vi "TLB Native Dynamic Events ver 0.26c.vi"() -> ()   [LabVIEW 2018] (continued)
                n641 = case shown="True" w1877 {
                  tunnel: [w1886 w1892] -> w1882
                  tunnel: w1878 -> [w1884 w1890]
                  frame False {
                    n642 = for {
                      tunnel: string[] ["CLOSE CLAW", "START TIMER"] ("element") -> [w1887] mode=indexing
                      shift-right: [w1889] -> w1886
                      shift-left: w1884 -> [w1888]
                      n643 = Enqueue Element(queue=w1888, element=w1887) -> (queue out=w1889:refnum<queue>)  [unwired: 2 in, 2 out]
                    }
                  }
                  frame True {
                    n644 = for {
                      shift-right: [w1894] -> w1892
                      shift-left: w1890 -> [w1895]
                      tunnel: string[] ["READ STEPPER VALUES", "", ""] -> [w1893] mode=indexing
                      n645 = Enqueue Element(queue=w1895, element=w1893) -> (queue out=w1894:refnum<queue>)  [unwired: 2 in, 2 out]
                    }
                  }
                }
                n646 = Or(x=w1877, y=w1873) -> (x .or. y?=w1880:bool)
                n647 = Select(t=State_Type_Definitions,_for_0.26g_versions_and_later_2."True Stop" ("Enum"), s=w1873, f=State_Type_Definitions,_for_0.26g_versions_and_later_2."Task 8K: RAISE MY SWORD" ("Enum")) -> (s? t:f=w1875:T18)
                n648 = Select(t=w1875, s=w1880, f=State_Type_Definitions,_for_0.26g_versions_and_later_2."Task 8J: CLOSE CLAW" ("Enum")) -> (s? t:f=w1879:T18)
              }
              frame "Exit" {
                n649 = for {
                  shift-right: [w1902] -> w1899
                  shift-left: w1896 -> [w1903]
                  tunnel: string[] ["STOP", "RESET ENCODERS", "RESET YAW", "ARDUINO MODE 0"] -> [w1901] mode=indexing
                  n650 = Enqueue Element(queue=w1903, element=w1901) -> (queue out=w1902:refnum<queue>)  [unwired: 2 in, 2 out]
                }
              }
            }
          }
          frame 37 {
            # ">>> yStepper command>>>"
            # ">> Manual override >>"
            n651 = Dequeue Element(queue=w1914, timeout in ms (-1)=w1913, error in (no error)=w1915) -> (element=w1912:T10)  [unwired: 3 out]
            n652 = Equal?(x=w1911, y=u8 60) -> (x = y?=w1909:bool)
            n653 = case shown="\"Start Task 1\", Default" w1912 {
              tunnel: [w1925 State_Type_Definitions,_for_0.26g_versions_and_later_2."True Stop" ("Enum")] -> w1916
              tunnel: [w1928 w1945] -> w1917
              tunnel: [State_Type_Definitions,_for_0.26g_versions_and_later_2."Idle" ("Enum") State_Type_Definitions,_for_0.26g_versions_and_later_2."Shutdown" ("Enum")] -> w1918
              tunnel: w1909 -> [w1924 _]
              tunnel: w1908 -> [w1923 _]
              tunnel: w1907 -> [w1919 w1942]
              frame "Start Task 1", Default {
                # "Stays in Task 5_A until stepper reaches desired \nheight"
                # "T: Go back to idle, F: Continue with task\""
                # ">> Manual override >>"
                n654 = case shown="True" w1924 {
                  tunnel: [w1932 w1938] -> w1928
                  tunnel: w1919 -> [w1930 w1936]
                  frame False {
                    n655 = for {
                      tunnel: string[] ["Z STEPPER CAM HEIGHT", "READ STEPPER VALUES"] ("element") -> [w1933] mode=indexing
                      shift-right: [w1935] -> w1932
                      shift-left: w1930 -> [w1934]
                      n656 = Enqueue Element(queue=w1934, element=w1933) -> (queue out=w1935:refnum<queue>)  [unwired: 2 in, 2 out]
                    }
                  }
                  frame True {
                    n657 = for {
                      shift-right: [w1940] -> w1938
                      shift-left: w1936 -> [w1941]
                      tunnel: string[] ["CAM CLOSE", "DISPOSE CAM BUFFERS", "DISPOSE PROC BUFFERS", "RESET ENCODERS"] -> [w1939] mode=indexing
                      n658 = Enqueue Element(queue=w1941, element=w1939) -> (queue out=w1940:refnum<queue>)  [unwired: 2 in, 2 out]
                    }
                  }
                }
                n659 = Or(x=w1924, y=w1923) -> (x .or. y?=w1926:bool)
                n660 = Select(t=State_Type_Definitions,_for_0.26g_versions_and_later_2."True Stop" ("Enum"), s=w1923, f=State_Type_Definitions,_for_0.26g_versions_and_later_2."True Stop" ("Enum")) -> (s? t:f=w1920:T18)
                n661 = Select(t=w1920, s=w1926, f=State_Type_Definitions,_for_0.26g_versions_and_later_2."Task 8K: RAISE MY SWORD" ("Enum")) -> (s? t:f=w1925:T18)
              }
              frame "Exit" {
                n662 = for {
                  shift-right: [w1948] -> w1945
                  shift-left: w1942 -> [w1949]
                  tunnel: string[] ["STOP", "RESET ENCODERS", "RESET YAW", "ARDUINO MODE 0"] -> [w1947] mode=indexing
                  n663 = Enqueue Element(queue=w1949, element=w1947) -> (queue out=w1948:refnum<queue>)  [unwired: 2 in, 2 out]
                }
              }
            }
          }
          frame 38 {
            # ">>> Motor control cluster >>>"
            # ">> Stepper height reeached >>"
            # ">>> yStepper command>>>"
            # ">> Manual override >>"
            n664 = Dequeue Element(queue=w1961, timeout in ms (-1)=w1956, error in (no error)=w1960) -> (element=w1964:T10)  [unwired: 3 out]
            n665 = Equal?(x=w1958, y=u8 40) -> (x = y?=w1962:bool)
            n666 = case shown="\"Start Task 1\", Default" w1964 {
              tunnel: [w1975 State_Type_Definitions,_for_0.26g_versions_and_later_2."True Stop" ("Enum")] -> w1954
              tunnel: [w1973 w1990] -> w1953
              tunnel: w1957 -> [w1972 _]
              tunnel: w1959 -> [w1966 _]
              tunnel: [State_Type_Definitions,_for_0.26g_versions_and_later_2."Idle" ("Enum") State_Type_Definitions,_for_0.26g_versions_and_later_2."Shutdown" ("Enum")] -> w1955
              tunnel: w1962 -> [w1965 _]
              frame "Start Task 1", Default {
                # ">> WIill proceed to part ii if not manual override >>"
                # ">>If ENABLE or Trigger is set to true>>"
                n667 = Or(x=w1965, y=w1966) -> (x .or. y?=w1967:bool)
                n668 = case shown="True" w1965 {
                  tunnel: [w1978 w1984] -> w1973
                  tunnel: w1972 -> [w1977 w1983]
                  frame False {
                    n669 = for {
                      shift-right: [w1980] -> w1978
                      shift-left: w1977 -> [w1981]
                      tunnel: string[] ["Z STEPPER BOX HEIGHT", "READ STEPPER VALUES"] ("element") -> [w1979] mode=indexing
                      n670 = Enqueue Element(queue=w1981, element=w1979) -> (queue out=w1980:refnum<queue>)  [unwired: 2 in, 2 out]
                    }
                  }
                  frame True {
                    n671 = for {
                      shift-right: [w1986] -> w1984
                      shift-left: w1983 -> [w1987]
                      tunnel: string[] ["OPEN LIFE CAM", "SET TIMER 5", "", "", "", ""] -> [w1985] mode=indexing
                      n672 = Enqueue Element(queue=w1987, element=w1985) -> (queue out=w1986:refnum<queue>)  [unwired: 2 in, 2 out]
                    }
                  }
                }
                n673 = Select(t=State_Type_Definitions,_for_0.26g_versions_and_later_2."True Stop" ("Enum"), s=w1966, f=State_Type_Definitions."Task 9F: SCAN IMAGE" ("Enum")) -> (s? t:f=w1969:u16)
                n674 = Select(t=w1969, s=w1967, f=State_Type_Definitions,_for_0.26g_versions_and_later_2."Task 9A: Raise Arm" ("Enum")) -> (s? t:f=w1975:u16)
              }
              frame "Exit" {
                n675 = for {
                  shift-right: [w1993] -> w1990
                  shift-left: _ -> [w1994]
                  tunnel: string[] ["STOP", "RESET ENCODERS", "RESET YAW", ""] -> [w1992] mode=indexing
                  n676 = Enqueue Element(queue=w1994, element=w1992) -> (queue out=w1993:refnum<queue>)  [unwired: 2 in, 2 out]
                }
              }
            }
          }
          frame 39 {
            # ">>> Motor control cluster >>>"
            # ">>> yStepper command>>>"
            n677 = Dequeue Element(queue=w2008, timeout in ms (-1)=w2007, error in (no error)=w2006) -> (element=w2010:T10)  [unwired: 3 out]
            n678 = In Range and Coerce(upper limit=65.0, x=w2000, lower limit=58.0) -> (In Range?=w1997:bool)  [unwired: 1 out]
            n679 = case shown="\"Start Task 1\", Default" w2010 {
              tunnel: w2001 -> [w2013 _]
              tunnel: [w2021 State_Type_Definitions,_for_0.26g_versions_and_later_2."True Stop" ("Enum")] -> w2003
              tunnel: w2009 -> [w2019 w2037]
              tunnel: [w2018 w2036] -> w2002
              tunnel: [State_Type_Definitions,_for_0.26g_versions_and_later_2."Idle" ("Enum") State_Type_Definitions,_for_0.26g_versions_and_later_2."Shutdown" ("Enum")] -> w2004
              tunnel: w1997 -> [w2011 _]
              frame "Start Task 1", Default {
                n680 = Or(x=w2011, y=w2013) -> (x .or. y?=w2012:bool)
                n681 = case shown="True" w2011 {
                  tunnel: w2019 -> [w2024 w2030]
                  tunnel: [w2023 w2028] -> w2018
                  frame False {
                    n682 = for {
                      shift-right: [w2026] -> w2023
                      shift-left: w2024 -> [w2027]
                      tunnel: string[] ["READ NAVX", "R-CW", "READ ULTRASONIC"] ("element") -> [w2025] mode=indexing
                      n683 = Enqueue Element(queue=w2027, element=w2025) -> (queue out=w2026:refnum<queue>)  [unwired: 2 in, 2 out]
                    }
                  }
                  frame True {
                    n684 = for {
                      shift-right: [w2032] -> w2028
                      shift-left: w2030 -> [w2033]
                      tunnel: string[] ["STOP", "RESET ENCODERS", "RESET YAW", "ARDUINO - ULTRASONIC", ""] -> [w2031] mode=indexing
                      n685 = Enqueue Element(queue=w2033, element=w2031) -> (queue out=w2032:refnum<queue>)  [unwired: 2 in, 2 out]
                    }
                  }
                }
                n686 = Select(t=State_Type_Definitions,_for_0.26g_versions_and_later_2."True Stop" ("Enum"), s=w2013, f=State_Type_Definitions,_for_0.26g_versions_and_later_2."Task 9C: Detect Box") -> (s? t:f=w2015:T18)
                n687 = Select(t=w2015, s=w2012, f=State_Type_Definitions,_for_0.26g_versions_and_later_2."Task 9B: Rotate to Angle" ("Enum")) -> (s? t:f=w2021:T18)
              }
              frame "Exit" {
                n688 = for {
                  shift-right: [w2040] -> w2036
                  shift-left: w2037 -> [w2041]
                  tunnel: string[] ["STOP", "RESET ENCODERS", "RESET YAW", ""] -> [w2039] mode=indexing
                  n689 = Enqueue Element(queue=w2041, element=w2039) -> (queue out=w2040:refnum<queue>)  [unwired: 2 in, 2 out]
                }
              }
            }
          }
          frame 40 {
            # ">>> Motor control cluster >>>"
            # ">>Line Detected>>"
            # ">>Action Queue>>"
            # ">>> yStepper command>>>"
            n690 = Dequeue Element(queue=w2053, timeout in ms (-1)=w2052, error in (no error)=w2051) -> (element=w2054:T10)  [unwired: 3 out]
            n691 = case shown="\"Start Task 1\", Default" w2054 {
              tunnel: w2049 -> [w2055 _]
              tunnel: [w2065 State_Type_Definitions,_for_0.26g_versions_and_later_2."True Stop" ("Enum")] -> w2046
              tunnel: w2050 -> [w2063 w2081]
              tunnel: [w2062 w2080] -> w2045
              tunnel: [State_Type_Definitions,_for_0.26g_versions_and_later_2."Idle" ("Enum") State_Type_Definitions,_for_0.26g_versions_and_later_2."Shutdown" ("Enum")] -> w2048
              tunnel: w2043 -> [w2056 _]
              frame "Start Task 1", Default {
                n692 = Or(x=w2055, y=w2056) -> (x .or. y?=w2057:bool)
                n693 = case shown="True" w2056 {
                  tunnel: w2063 -> [w2068 w2074]
                  tunnel: [w2067 w2072] -> w2062
                  frame False {
                    n694 = for {
                      shift-right: [w2070] -> w2067
                      shift-left: w2068 -> [w2071]
                      tunnel: string[] ["READ IR", "READ LINE SENSOR", "FORWARD - IR ASSIST"] ("element") -> [w2069] mode=indexing
                      n695 = Enqueue Element(queue=w2071, element=w2069) -> (queue out=w2070:refnum<queue>)  [unwired: 2 in, 2 out]
                    }
                  }
                  frame True {
                    n696 = for {
                      shift-right: [w2076] -> w2072
                      shift-left: w2074 -> [w2077]
                      tunnel: string[] ["STOP", "RESET ENCODERS", "RESET YAW", ""] -> [w2075] mode=indexing
                      n697 = Enqueue Element(queue=w2077, element=w2075) -> (queue out=w2076:refnum<queue>)  [unwired: 2 in, 2 out]
                    }
                  }
                }
                n698 = Select(t=State_Type_Definitions,_for_0.26g_versions_and_later_2."True Stop" ("Enum"), s=w2055, f=State_Type_Definitions,_for_0.26g_versions_and_later_2."Task 9D: MOVE FORWARD") -> (s? t:f=w2059:T18)
                n699 = Select(t=w2059, s=w2057, f=State_Type_Definitions,_for_0.26g_versions_and_later_2."Task 9C: Detect Box" ("Enum")) -> (s? t:f=w2065:T18)
              }
              frame "Exit" {
                n700 = for {
                  shift-right: [w2084] -> w2080
                  shift-left: w2081 -> [w2085]
                  tunnel: string[] ["STOP", "RESET ENCODERS", "RESET YAW", ""] -> [w2083] mode=indexing
                  n701 = Enqueue Element(queue=w2085, element=w2083) -> (queue out=w2084:refnum<queue>)  [unwired: 2 in, 2 out]
                }
              }
            }
          }
          frame 41 {
            (unwired) 50.0 ("y")
            # ">> Item Selection Bias >>"
            # ">> Wall detected >>"
            # ">> Manual override >>"
            # ">>Table Detected>>"
            # ">>> Motor control cluster >>>"
            # ">>Table or wall detectected>>"
            # ">>Action Queue>>"
            # ">>> yStepper command>>>"
            n702 = Dequeue Element(queue=w2103, timeout in ms (-1)=w2102, error in (no error)=w2101) -> (element=w2104:T10)  [unwired: 3 out]
            n703 = Less Or Equal?(x=w2092, y=20.0) -> (x <= y?=w2087:bool)
            n704 = Less?(x=w2090, y=20.0) -> (x < y?=w2088:bool)
            n705 = Or(x=w2087, y=w2088) -> (x .or. y?=w2086:bool)
            n706 = case shown="\"Start Task 1\", Default" w2104 {
              tunnel: w2099 -> [w2105 _]
              tunnel: [w2115 State_Type_Definitions,_for_0.26g_versions_and_later_2."True Stop" ("Enum")] -> w2096
              tunnel: w2100 -> [w2113 w2131]
              tunnel: [w2112 w2130] -> w2095
              tunnel: [State_Type_Definitions,_for_0.26g_versions_and_later_2."Idle" ("Enum") State_Type_Definitions,_for_0.26g_versions_and_later_2."Shutdown" ("Enum")] -> w2098
              tunnel: w2086 -> [w2106 _]
              frame "Start Task 1", Default {
                n707 = Or(x=w2105, y=w2106) -> (x .or. y?=w2107:bool)
                n708 = case shown="True" w2106 {
                  tunnel: w2113 -> [w2118 w2124]
                  tunnel: [w2117 w2122] -> w2112
                  frame False {
                    n709 = for {
                      shift-right: [w2120] -> w2117
                      shift-left: w2118 -> [w2121]
                      tunnel: string[] ["READ IR", "FORWARD - IR ASSIST", "READ ULTRASONIC"] ("element") -> [w2119] mode=indexing
                      n710 = Enqueue Element(queue=w2121, element=w2119) -> (queue out=w2120:refnum<queue>)  [unwired: 2 in, 2 out]
                    }
                  }
                  frame True {
                    n711 = for {
                      shift-right: [w2126] -> w2122
                      shift-left: w2124 -> [w2127]
                      tunnel: string[] ["STOP", "RESET ENCODERS", "RESET YAW", ""] -> [w2125] mode=indexing
                      n712 = Enqueue Element(queue=w2127, element=w2125) -> (queue out=w2126:refnum<queue>)  [unwired: 2 in, 2 out]
                    }
                  }
                }
                n713 = Select(t=State_Type_Definitions,_for_0.26g_versions_and_later_2."True Stop" ("Enum"), s=w2105, f=State_Type_Definitions,_for_0.26g_versions_and_later_2."Task 9E: MOVE LEFT") -> (s? t:f=w2109:T18)
                n714 = Select(t=w2109, s=w2107, f=State_Type_Definitions,_for_0.26g_versions_and_later_2."Task 9D: MOVE FORWARD" ("Enum")) -> (s? t:f=w2115:T18)
              }
              frame "Exit" {
                n715 = for {
                  shift-right: [w2134] -> w2130
                  shift-left: w2131 -> [w2135]
                  tunnel: string[] ["STOP", "RESET ENCODERS", "RESET YAW", ""] -> [w2133] mode=indexing
                  n716 = Enqueue Element(queue=w2135, element=w2133) -> (queue out=w2134:refnum<queue>)  [unwired: 2 in, 2 out]
                }
              }
            }
          }
          frame 42 {
            # ">> Item Selection Bias >>"
            # ">> Line detected? >>"
            # ">> Manual override >>"
            # ">>> Motor control cluster >>>"
            # ">>Action Queue>>"
            # ">>> yStepper command>>>"
            n717 = Dequeue Element(queue=w2147, timeout in ms (-1)=w2146, error in (no error)=w2145) -> (element=w2148:T10)  [unwired: 3 out]
            n718 = case shown="\"Start Task 1\", Default" w2148 {
              tunnel: w2143 -> [w2149 _]
              tunnel: [w2159 State_Type_Definitions,_for_0.26g_versions_and_later_2."True Stop" ("Enum")] -> w2140
              tunnel: w2144 -> [w2157 w2175]
              tunnel: [w2156 w2174] -> w2139
              tunnel: [State_Type_Definitions,_for_0.26g_versions_and_later_2."Idle" ("Enum") State_Type_Definitions,_for_0.26g_versions_and_later_2."Shutdown" ("Enum")] -> w2142
              tunnel: w2136 -> [w2150 _]
              frame "Start Task 1", Default {
                n719 = Or(x=w2149, y=w2150) -> (x .or. y?=w2151:bool)
                n720 = case shown="True" w2150 {
                  tunnel: w2157 -> [w2162 w2168]
                  tunnel: [w2161 w2166] -> w2156
                  frame False {
                    n721 = for {
                      shift-right: [w2164] -> w2161
                      shift-left: w2162 -> [w2165]
                      tunnel: string[] ["LEFT", "READ NAVX", "READ LINE SENSOR", ""] ("element") -> [w2163] mode=indexing
                      n722 = Enqueue Element(queue=w2165, element=w2163) -> (queue out=w2164:refnum<queue>)  [unwired: 2 in, 2 out]
                    }
                  }
                  frame True {
                    n723 = for {
                      shift-right: [w2170] -> w2166
                      shift-left: w2168 -> [w2171]
                      tunnel: string[] ["STOP", "RESET ENCODERS", "RESET YAW", "RESET FLAGS", "OPEN LIFE CAM", "SET TIMER 2"] -> [w2169] mode=indexing
                      n724 = Enqueue Element(queue=w2171, element=w2169) -> (queue out=w2170:refnum<queue>)  [unwired: 2 in, 2 out]
                    }
                  }
                }
                n725 = Select(t=State_Type_Definitions,_for_0.26g_versions_and_later_2."True Stop" ("Enum"), s=w2149, f=State_Type_Definitions."Task 9F: SCAN IMAGE") -> (s? t:f=w2153:u16)
                n726 = Select(t=w2153, s=w2151, f=State_Type_Definitions,_for_0.26g_versions_and_later_2."Task 9E: MOVE LEFT" ("Enum")) -> (s? t:f=w2159:u16)
              }
              frame "Exit" {
                n727 = for {
                  shift-right: [w2178] -> w2174
                  shift-left: w2175 -> [w2179]
                  tunnel: string[] ["STOP", "RESET ENCODERS", "RESET YAW", ""] -> [w2177] mode=indexing
                  n728 = Enqueue Element(queue=w2179, element=w2177) -> (queue out=w2178:refnum<queue>)  [unwired: 2 in, 2 out]
                }
              }
            }
          }
          frame 43 {
            # ">>> Motor control cluster >>>"
            # ">>Time up? >>"
            # ">>> yStepper command>>>"
            # ">> Manual override >>"
            n729 = Dequeue Element(queue=w2191, timeout in ms (-1)=w2187, error in (no error)=w2190) -> (element=w2192:T10)  [unwired: 3 out]
            n730 = case shown="\"Start Task 1\", Default" w2192 {
              tunnel: [w2203 State_Type_Definitions,_for_0.26g_versions_and_later_2."True Stop" ("Enum")] -> w2185
              tunnel: [w2201 w2219] -> w2184
              tunnel: w2188 -> [w2200 w2216]
              tunnel: w2189 -> [w2194 _]
              tunnel: [State_Type_Definitions,_for_0.26g_versions_and_later_2."Idle" ("Enum") State_Type_Definitions,_for_0.26g_versions_and_later_2."Shutdown" ("Enum")] -> w2186
              tunnel: w2180 -> [w2193 _]
              frame "Start Task 1", Default {
                # ">> WIill proceed to part ii if not manual override >>"
                # ">>If ENABLE or Trigger is set to true>>"
                n731 = Or(x=w2193, y=w2194) -> (x .or. y?=w2195:bool)
                n732 = case shown="True" w2193 {
                  tunnel: [w2206 w2212] -> w2201
                  tunnel: w2200 -> [w2205 w2211]
                  frame False {
                    n733 = for {
                      shift-right: [w2208] -> w2206
                      shift-left: w2205 -> [w2209]
                      tunnel: string[] ["CAM ACQ", "START TIMER"] ("element") -> [w2207] mode=indexing
                      n734 = Enqueue Element(queue=w2209, element=w2207) -> (queue out=w2208:refnum<queue>)  [unwired: 2 in, 2 out]
                    }
                  }
                  frame True {
                    n735 = for {
                      shift-right: [w2214] -> w2212
                      shift-left: w2211 -> [w2215]
                      tunnel: string[] ["CLOSE CAM", "SET TIMER 2", "RESET FLAGS", "", "", ""] -> [w2213] mode=indexing
                      n736 = Enqueue Element(queue=w2215, element=w2213) -> (queue out=w2214:refnum<queue>)  [unwired: 2 in, 2 out]
                    }
                  }
                }
                n737 = Select(t=State_Type_Definitions,_for_0.26g_versions_and_later_2."True Stop" ("Enum"), s=w2194, f=State_Type_Definitions."Task 9G: PROCESS COLOUR" ("Enum")) -> (s? t:f=w2197:u16)
                n738 = Select(t=w2197, s=w2195, f=State_Type_Definitions."Task 9F: SCAN IMAGE" ("Enum")) -> (s? t:f=w2203:u16)
              }
              frame "Exit" {
                n739 = for {
                  shift-right: [w2222] -> w2219
                  shift-left: w2216 -> [w2223]
                  tunnel: string[] ["STOP", "RESET ENCODERS", "RESET YAW", ""] -> [w2221] mode=indexing
                  n740 = Enqueue Element(queue=w2223, element=w2221) -> (queue out=w2222:refnum<queue>)  [unwired: 2 in, 2 out]
                }
              }
            }
          }
          frame 44 {
            # ">>> Motor control cluster >>>"
            # ">>> yStepper command>>>"
            n741 = Dequeue Element(queue=w2231, timeout in ms (-1)=w2230, error in (no error)=w2229) -> (element=w2236:T10)  [unwired: 3 out]
            n742 = case shown="\"Start Task 1\", Default" w2236 {
              tunnel: w2224 -> [w2239 _]
              tunnel: [w2246 State_Type_Definitions,_for_0.26g_versions_and_later_2."True Stop" ("Enum")] -> w2235
              tunnel: w2228 -> [w2238 _]
              tunnel: w2232 -> [w2245 w2262]
              tunnel: [w2244 w2263] -> w2234
              tunnel: [State_Type_Definitions,_for_0.26g_versions_and_later_2."Idle" ("Enum") State_Type_Definitions,_for_0.26g_versions_and_later_2."Shutdown" ("Enum")] -> w2233
              frame "Start Task 1", Default {
                n743 = case shown="False" w2239 {
                  tunnel: w2245 -> [w2249 w2256]
                  tunnel: [w2250 w2255] -> w2244
                  frame False {
                    n744 = for {
                      tunnel: string[] ["START TIMER", "COLOUR PROCESSING", ""] ("element") -> [w2251] mode=indexing
                      shift-right: [w2253] -> w2250
                      shift-left: w2249 -> [w2252]
                      n745 = Enqueue Element(queue=w2252, element=w2251) -> (queue out=w2253:refnum<queue>)  [unwired: 2 in, 2 out]
                    }
                  }
                  frame True {
                    n746 = for {
                      shift-right: [w2258] -> w2255
                      shift-left: w2256 -> [w2259]
                      tunnel: string[] ["DISPOSE BUFFERS", "CLOSE CAM", "RESET ENCODERS", "RESET YAW", "RESET FLAGS"] -> [w2257] mode=indexing
                      n747 = Enqueue Element(queue=w2259, element=w2257) -> (queue out=w2258:refnum<queue>)  [unwired: 2 in, 2 out]
                    }
                  }
                }
                n748 = Or(x=w2239, y=w2238) -> (x .or. y?=w2237:bool)
                n749 = Select(t=State_Type_Definitions,_for_0.26g_versions_and_later_2."True Stop" ("Enum"), s=w2238, f=State_Type_Definitions,_for_0.26g_versions_and_later_2."True Stop" ("Enum")) -> (s? t:f=w2240:T18)
                n750 = Select(t=w2240, s=w2237, f=State_Type_Definitions."Task 9G: PROCESS COLOUR" ("Enum")) -> (s? t:f=w2246:u16)
              }
              frame "Exit" {
                n751 = for {
                  shift-right: [w2266] -> w2263
                  shift-left: w2262 -> [w2267]
                  tunnel: string[] ["STOP", "RESET ENCODERS", "RESET YAW", "ARDUINO MODE 0"] -> [w2265] mode=indexing
                  n752 = Enqueue Element(queue=w2267, element=w2265) -> (queue out=w2266:refnum<queue>)  [unwired: 2 in, 2 out]
                }
              }
            }
          }
          frame 45 {
            # ">> Item Selection Bias >>"
            # ">>> Motor control cluster >>>"
            # ">>> yStepper command>>>"
            n753 = Dequeue Element(queue=w2277, timeout in ms (-1)=w2278, error in (no error)=w2279) -> (element=w2281:T10)  [unwired: 3 out]
            n754 = Greater?(x=w2269, y=50.0) -> (0:w2270:bool)
            n755 = And(x=w2271, y=w2270) -> (x .and. y?=w2272:bool)
            n756 = case shown="\"Start Task 1\", Default" w2281 {
              tunnel: w2272 -> [w2287 _]
              tunnel: [w2294 State_Type_Definitions,_for_0.26g_versions_and_later_2."True Stop" ("Enum")] -> w2274
              tunnel: w2280 -> [w2286 _]
              tunnel: w2276 -> [w2293 w2310]
              tunnel: [w2292 w2311] -> w2275
              tunnel: [State_Type_Definitions,_for_0.26g_versions_and_later_2."Idle" ("Enum") State_Type_Definitions,_for_0.26g_versions_and_later_2."Shutdown" ("Enum")] -> w2273
              frame "Start Task 1", Default {
                n757 = case shown="True" w2287 {
                  tunnel: w2293 -> [w2297 w2304]
                  tunnel: [w2298 w2303] -> w2292
                  frame False {
                    n758 = for {
                      tunnel: string[] ["READ LINE SENSOR", "READ NAVX", "RIGHT", "READ ENCODERS"] ("element") -> [w2299] mode=indexing
                      shift-right: [w2301] -> w2298
                      shift-left: w2297 -> [w2300]
                      n759 = Enqueue Element(queue=w2300, element=w2299) -> (queue out=w2301:refnum<queue>)  [unwired: 2 in, 2 out]
                    }
                  }
                  frame True {
                    n760 = for {
                      shift-right: [w2306] -> w2303
                      shift-left: w2304 -> [w2307]
                      tunnel: string[] ["STOP", "RESET ENCODERS", "RESET YAW", "OPEN LIFE CAM", "SET TIMER 5", "RESET FLAGS"] -> [w2305] mode=indexing
                      n761 = Enqueue Element(queue=w2307, element=w2305) -> (queue out=w2306:refnum<queue>)  [unwired: 2 in, 2 out]
                    }
                  }
                }
                n762 = Or(x=w2287, y=w2286) -> (x .or. y?=w2285:bool)
                n763 = Select(t=State_Type_Definitions,_for_0.26g_versions_and_later_2."True Stop" ("Enum"), s=w2286, f=State_Type_Definitions,_for_0.26d_versions_and_later."Task 9I: SCAN IMAGE" ("Enum")) -> (s? t:f=w2288:u16)
                n764 = Select(t=w2288, s=w2285, f=State_Type_Definitions."Task 9H: MOVE RIGHT" ("Enum")) -> (s? t:f=w2294:u16)
              }
              frame "Exit" {
                n765 = for {
                  shift-right: [w2314] -> w2311
                  shift-left: w2310 -> [w2315]
                  tunnel: string[] ["STOP", "RESET ENCODERS", "RESET YAW", "ARDUINO MODE 0"] -> [w2313] mode=indexing
                  n766 = Enqueue Element(queue=w2315, element=w2313) -> (queue out=w2314:refnum<queue>)  [unwired: 2 in, 2 out]
                }
              }
            }
          }
          frame 46 {
            # ">> Item Selection Bias >>"
            n767 = Dequeue Element(queue=w2317, timeout in ms (-1)=w2318, error in (no error)=w2319) -> (element=w2325:T10)  [unwired: 3 out]
            n768 = case shown="\"Start Task 1\", Default" w2325 {
              tunnel: w2316 -> [w2331 _]
              tunnel: [w2338 State_Type_Definitions,_for_0.26g_versions_and_later_2."True Stop" ("Enum")] -> w2322
              tunnel: w2320 -> [w2330 _]
              tunnel: w2324 -> [w2337 w2354]
              tunnel: [w2336 w2355] -> w2323
              tunnel: [State_Type_Definitions,_for_0.26g_versions_and_later_2."Idle" ("Enum") State_Type_Definitions,_for_0.26g_versions_and_later_2."Shutdown" ("Enum")] -> w2321
              frame "Start Task 1", Default {
                n769 = case shown="True" w2331 {
                  tunnel: w2337 -> [w2341 w2348]
                  tunnel: [w2342 w2347] -> w2336
                  frame False {
                    n770 = for {
                      tunnel: string[] ["START TIMER", "CAM ACQ", ""] ("element") -> [w2343] mode=indexing
                      shift-right: [w2345] -> w2342
                      shift-left: w2341 -> [w2344]
                      n771 = Enqueue Element(queue=w2344, element=w2343) -> (queue out=w2345:refnum<queue>)  [unwired: 2 in, 2 out]
                    }
                  }
                  frame True {
                    n772 = for {
                      shift-right: [w2350] -> w2347
                      shift-left: w2348 -> [w2351]
                      tunnel: string[] ["CLOSE CAM", "SET TIMER 5", "", "", "", ""] -> [w2349] mode=indexing
                      n773 = Enqueue Element(queue=w2351, element=w2349) -> (queue out=w2350:refnum<queue>)  [unwired: 2 in, 2 out]
                    }
                  }
                }
                n774 = Or(x=w2331, y=w2330) -> (x .or. y?=w2329:bool)
                n775 = Select(t=State_Type_Definitions,_for_0.26g_versions_and_later_2."True Stop" ("Enum"), s=w2330, f=State_Type_Definitions,_for_0.26d_versions_and_later."Task 9J: PROCESS COLOUR" ("Enum")) -> (s? t:f=w2332:u16)
                n776 = Select(t=w2332, s=w2329, f=State_Type_Definitions,_for_0.26d_versions_and_later."Task 9I: SCAN IMAGE" ("Enum")) -> (s? t:f=w2338:u16)
              }
              frame "Exit" {
                n777 = for {
                  shift-right: [w2358] -> w2355
                  shift-left: w2354 -> [w2359]
                  tunnel: string[] ["STOP", "RESET ENCODERS", "RESET YAW", "ARDUINO MODE 0"] -> [w2357] mode=indexing
                  n778 = Enqueue Element(queue=w2359, element=w2357) -> (queue out=w2358:refnum<queue>)  [unwired: 2 in, 2 out]
                }
              }
            }
          }
          frame 47 {
            # ">> Item Selection Bias >>"
            n779 = Dequeue Element(queue=w2365, timeout in ms (-1)=w2366, error in (no error)=w2367) -> (element=w2369:T10)  [unwired: 3 out]
            n780 = case shown="\"Start Task 1\", Default" w2369 {
              tunnel: w2360 -> [w2375 _]
              tunnel: [w2382 State_Type_Definitions,_for_0.26g_versions_and_later_2."True Stop" ("Enum")] -> w2363
              tunnel: w2368 -> [w2374 _]
              tunnel: w2364 -> [w2381 w2398]
              tunnel: [w2380 w2399] -> w2362
              tunnel: [State_Type_Definitions,_for_0.26g_versions_and_later_2."Idle" ("Enum") State_Type_Definitions,_for_0.26g_versions_and_later_2."Shutdown" ("Enum")] -> w2361
              frame "Start Task 1", Default {
                n781 = case shown="True" w2375 {
                  tunnel: w2381 -> [w2385 w2392]
                  tunnel: [w2386 w2391] -> w2380
                  frame False {
                    n782 = for {
                      tunnel: string[] ["START TIMER", "COLOUR PROCESSING", ""] ("element") -> [w2387] mode=indexing
                      shift-right: [w2389] -> w2386
                      shift-left: w2385 -> [w2388]
                      n783 = Enqueue Element(queue=w2388, element=w2387) -> (queue out=w2389:refnum<queue>)  [unwired: 2 in, 2 out]
                    }
                  }
                  frame True {
                    n784 = for {
                      shift-right: [w2394] -> w2391
                      shift-left: w2392 -> [w2395]
                      tunnel: string[] ["CLOSE CAM", "DISPOSE BUFFERS", "RESET ENCODERS", "RESET YAW", "RESET FLAGS", ""] -> [w2393] mode=indexing
                      n785 = Enqueue Element(queue=w2395, element=w2393) -> (queue out=w2394:refnum<queue>)  [unwired: 2 in, 2 out]
                    }
                  }
                }
                n786 = Or(x=w2375, y=w2374) -> (x .or. y?=w2373:bool)
                n787 = Select(t=State_Type_Definitions,_for_0.26g_versions_and_later_2."True Stop" ("Enum"), s=w2374, f=State_Type_Definitions,_for_0.26g_versions_and_later_2."True Stop" ("Enum")) -> (s? t:f=w2376:T18)
                n788 = Select(t=w2376, s=w2373, f=State_Type_Definitions,_for_0.26d_versions_and_later."Task 9J: PROCESS COLOUR" ("Enum")) -> (s? t:f=w2382:u16)
              }
              frame "Exit" {
                n789 = for {
                  shift-right: [w2402] -> w2399
                  shift-left: w2398 -> [w2403]
                  tunnel: string[] ["STOP", "RESET ENCODERS", "RESET YAW", "ARDUINO MODE 0"] -> [w2401] mode=indexing
                  n790 = Enqueue Element(queue=w2403, element=w2401) -> (queue out=w2402:refnum<queue>)  [unwired: 2 in, 2 out]
                }
              }
            }
          }
          frame 48 {
            # ">>> Motor control cluster >>>"
            # ">>> yStepper command>>>"
            # ">> Item Selection Bias >>"
            n791 = Less?(x=w2407, y=-38.0) -> (x < y?=w2405:bool)
            n792 = Dequeue Element(queue=w2413, timeout in ms (-1)=w2412, error in (no error)=w2411) -> (element=w2415:T10)  [unwired: 3 out]
            n793 = case shown="\"Start Task 1\", Default" w2415 {
              tunnel: w2405 -> [w2421 _]
              tunnel: [w2428 State_Type_Definitions,_for_0.26g_versions_and_later_2."True Stop" ("Enum")] -> w2409
              tunnel: w2410 -> [w2420 _]
              tunnel: w2414 -> [w2427 w2444]
              tunnel: [w2426 w2445] -> w2404
              tunnel: [State_Type_Definitions,_for_0.26g_versions_and_later_2."Idle" ("Enum") State_Type_Definitions,_for_0.26g_versions_and_later_2."Shutdown" ("Enum")] -> w2408
              frame "Start Task 1", Default {
                n794 = case shown="True" w2421 {
                  tunnel: w2427 -> [w2431 w2438]
                  tunnel: [w2432 w2437] -> w2426
                  frame False {
                    n795 = for {
                      tunnel: string[] ["READ ENCODERS", "R-CW"] ("element") -> [w2433] mode=indexing
                      shift-right: [w2435] -> w2432
                      shift-left: w2431 -> [w2434]
                      n796 = Enqueue Element(queue=w2434, element=w2433) -> (queue out=w2435:refnum<queue>)  [unwired: 2 in, 2 out]
                    }
                  }
                  frame True {
                    n797 = for {
                      shift-right: [w2440] -> w2437
                      shift-left: w2438 -> [w2441]
                      tunnel: string[] ["STOP", "RESET ENCODERS", "RESET FLAGS", "RESET YAW", "READ IR", "ARDUINO - ULTRASONIC"] -> [w2439] mode=indexing
                      n798 = Enqueue Element(queue=w2441, element=w2439) -> (queue out=w2440:refnum<queue>)  [unwired: 2 in, 2 out]
                    }
                  }
                }
                n799 = Or(x=w2421, y=w2420) -> (x .or. y?=w2419:bool)
                n800 = Select(t=State_Type_Definitions,_for_0.26g_versions_and_later_2."True Stop" ("Enum"), s=w2420, f=State_Type_Definitions,_for_0.26d_versions_and_later."Task 9L: MOVE FORWARD" ("Enum")) -> (s? t:f=w2422:u16)
                n801 = Select(t=w2422, s=w2419, f=State_Type_Definitions,_for_0.26d_versions_and_later."Task 9K: ROTATE 90 CW" ("Enum")) -> (s? t:f=w2428:u16)
              }
              frame "Exit" {
                n802 = for {
                  shift-right: [w2448] -> w2445
                  shift-left: w2444 -> [w2449]
                  tunnel: string[] ["STOP", "RESET ENCODERS", "RESET YAW", "ARDUINO MODE 0"] -> [w2447] mode=indexing
                  n803 = Enqueue Element(queue=w2449, element=w2447) -> (queue out=w2448:refnum<queue>)  [unwired: 2 in, 2 out]
                }
              }
            }
          }
          frame 49 {
            w2462 = u8 50 ("y")
            # ">>> Motor control cluster >>>"
            # ">>> yStepper command>>>"
            # ">> Item Selection Bias >>"
            n804 = Less?(x=w2464, y=w2462) -> (x < y?=w2457:bool)
            n805 = Dequeue Element(queue=w2468, timeout in ms (-1)=w2467, error in (no error)=w2466) -> (element=w2472:T10)  [unwired: 3 out]
            n806 = Less?(x=w2463, y=w2462) -> (x < y?=w2458:bool)
            n807 = And(x=w2458, y=w2457) -> (x .and. y?=w2450:bool)
            n808 = Less Or Equal?(x=w2461, y=15.0) -> (x <= y?=w2456:bool)
            n809 = Greater?(x=w2455, y=100.0) -> (0:w2454:bool)
            n810 = Or(x=w2456, y=w2450) -> (x .or. y?=w2452:bool)
            n811 = And(x=w2454, y=w2452) -> (x .and. y?=w2453:bool)
            n812 = case shown="\"Start Task 1\", Default" w2472 {
              tunnel: w2453 -> [w2478 _]
              tunnel: [w2485 State_Type_Definitions,_for_0.26g_versions_and_later_2."True Stop" ("Enum")] -> w2470
              tunnel: w2465 -> [w2477 _]
              tunnel: w2469 -> [w2484 w2501]
              tunnel: [w2483 w2502] -> w2459
              tunnel: [State_Type_Definitions,_for_0.26g_versions_and_later_2."Idle" ("Enum") State_Type_Definitions,_for_0.26g_versions_and_later_2."Shutdown" ("Enum")] -> w2471
              frame "Start Task 1", Default {
                n813 = case shown="True" w2478 {
                  tunnel: w2484 -> [w2488 w2495]
                  tunnel: [w2489 w2494] -> w2483
                  frame False {
                    n814 = for {
                      tunnel: string[] ["READ IR", "FORWARD", "READ NAVX", "READ ENCODERS"] ("element") -> [w2490] mode=indexing
                      shift-right: [w2492] -> w2489
                      shift-left: w2488 -> [w2491]
                      n815 = Enqueue Element(queue=w2491, element=w2490) -> (queue out=w2492:refnum<queue>)  [unwired: 2 in, 2 out]
                    }
                  }
                  frame True {
                    n816 = for {
                      shift-right: [w2497] -> w2494
                      shift-left: w2495 -> [w2498]
                      tunnel: string[] ["STOP", "RESET ENCODERS", "RESET FLAGS", "RESET YAW", "", ""] -> [w2496] mode=indexing
                      n817 = Enqueue Element(queue=w2498, element=w2496) -> (queue out=w2497:refnum<queue>)  [unwired: 2 in, 2 out]
                    }
                  }
                }
                n818 = Or(x=w2478, y=w2477) -> (x .or. y?=w2476:bool)
                n819 = Select(t=State_Type_Definitions,_for_0.26g_versions_and_later_2."True Stop" ("Enum"), s=w2477, f=State_Type_Definitions,_for_0.26g_versions_and_later_2."True Stop" ("Enum")) -> (s? t:f=w2479:T18)
                n820 = Select(t=w2479, s=w2476, f=State_Type_Definitions,_for_0.26d_versions_and_later."Task 9L: MOVE FORWARD" ("Enum")) -> (s? t:f=w2485:u16)
              }
              frame "Exit" {
                n821 = for {
                  shift-right: [w2505] -> w2502
                  shift-left: w2501 -> [w2506]
                  tunnel: string[] ["STOP", "RESET ENCODERS", "RESET YAW", "ARDUINO MODE 0"] -> [w2504] mode=indexing
                  n822 = Enqueue Element(queue=w2506, element=w2504) -> (queue out=w2505:refnum<queue>)  [unwired: 2 in, 2 out]
                }
              }
            }
          }
          frame 50 {
            # ">> Item Selection Bias >>"
            n823 = Dequeue Element(queue=w2511, timeout in ms (-1)=w2510, error in (no error)=w2509) -> (element=w2516:T10)  [unwired: 3 out]
            n824 = case shown="\"Start Task 1\", Default" w2516 {
              tunnel: w2507 -> [w2522 _]
              tunnel: [w2529 State_Type_Definitions,_for_0.26g_versions_and_later_2."True Stop" ("Enum")] -> w2514
              tunnel: w2508 -> [w2521 _]
              tunnel: w2512 -> [w2528 w2545]
              tunnel: [w2527 w2546] -> w2513
              tunnel: [State_Type_Definitions,_for_0.26g_versions_and_later_2."Idle" ("Enum") State_Type_Definitions,_for_0.26g_versions_and_later_2."Shutdown" ("Enum")] -> w2515
              frame "Start Task 1", Default {
                n825 = case shown="False" w2522 {
                  tunnel: w2528 -> [w2532 w2539]
                  tunnel: [w2533 w2538] -> w2527
                  frame False {
                    n826 = for {
                      tunnel: string[] ["READ LINE SENSOR", "READ NAVX", "RIGHT", "READ ENCODERS"] ("element") -> [w2534] mode=indexing
                      shift-right: [w2536] -> w2533
                      shift-left: w2532 -> [w2535]
                      n827 = Enqueue Element(queue=w2535, element=w2534) -> (queue out=w2536:refnum<queue>)  [unwired: 2 in, 2 out]
                    }
                  }
                  frame True {
                    n828 = for {
                      shift-right: [w2541] -> w2538
                      shift-left: w2539 -> [w2542]
                      tunnel: string[] ["STOP", "RESET ENCODERS", "RESET YAW", "OPEN LIFE CAM", "SET TIMER 2", "RESET FLAGS"] -> [w2540] mode=indexing
                      n829 = Enqueue Element(queue=w2542, element=w2540) -> (queue out=w2541:refnum<queue>)  [unwired: 2 in, 2 out]
                    }
                  }
                }
                n830 = Or(x=w2522, y=w2521) -> (x .or. y?=w2520:bool)
                n831 = Select(t=State_Type_Definitions,_for_0.26g_versions_and_later_2."True Stop" ("Enum"), s=w2521, f=State_Type_Definitions,_for_0.26d_versions_and_later."Task 9N: SCAN IMAGE" ("Enum")) -> (s? t:f=w2523:u16)
                n832 = Select(t=w2523, s=w2520, f=State_Type_Definitions,_for_0.26g_versions_and_later_2."Task 9M: MOVE RIGHT" ("Enum")) -> (s? t:f=w2529:u16)
              }
              frame "Exit" {
                n833 = for {
                  shift-right: [w2549] -> w2546
                  shift-left: w2545 -> [w2550]
                  tunnel: string[] ["STOP", "RESET ENCODERS", "RESET YAW", "ARDUINO MODE 0"] -> [w2548] mode=indexing
                  n834 = Enqueue Element(queue=w2550, element=w2548) -> (queue out=w2549:refnum<queue>)  [unwired: 2 in, 2 out]
                }
              }
            }
          }
          frame 51 {
            # ">> Manual override >>"
            n835 = Dequeue Element(queue=w2559, timeout in ms (-1)=w2558, error in (no error)=w2557) -> (element=w2560:T10)  [unwired: 3 out]
            n836 = case shown="\"Start Task 1\", Default" w2560 {
              tunnel: [w2574 State_Type_Definitions,_for_0.26g_versions_and_later_2."True Stop" ("Enum")] -> w2552
              tunnel: [w2572 w2590] -> w2551
              tunnel: w2555 -> [w2571 w2587]
              tunnel: w2556 -> [w2565 _]
              tunnel: [State_Type_Definitions,_for_0.26g_versions_and_later_2."Idle" ("Enum") State_Type_Definitions,_for_0.26g_versions_and_later_2."Shutdown" ("Enum")] -> w2553
              tunnel: w2554 -> [w2564 _]
              frame "Start Task 1", Default {
                # ">> WIill proceed to part ii if not manual override >>"
                # ">>If ENABLE or Trigger is set to true>>"
                n837 = Or(x=w2564, y=w2565) -> (x .or. y?=w2566:bool)
                n838 = case shown="False" w2564 {
                  tunnel: [w2577 w2583] -> w2572
                  tunnel: w2571 -> [w2576 w2582]
                  frame False {
                    n839 = for {
                      shift-right: [w2579] -> w2577
                      shift-left: w2576 -> [w2580]
                      tunnel: string[] ["CAM ACQ", "START TIMER"] ("element") -> [w2578] mode=indexing
                      n840 = Enqueue Element(queue=w2580, element=w2578) -> (queue out=w2579:refnum<queue>)  [unwired: 2 in, 2 out]
                    }
                  }
                  frame True {
                    n841 = for {
                      shift-right: [w2585] -> w2583
                      shift-left: w2582 -> [w2586]
                      tunnel: string[] ["CLOSE CAM", "SET TIMER 5", "", "", "", ""] -> [w2584] mode=indexing
                      n842 = Enqueue Element(queue=w2586, element=w2584) -> (queue out=w2585:refnum<queue>)  [unwired: 2 in, 2 out]
                    }
                  }
                }
                n843 = Select(t=State_Type_Definitions,_for_0.26g_versions_and_later_2."True Stop" ("Enum"), s=w2565, f=State_Type_Definitions,_for_0.26d_versions_and_later."Task 9O: PROCESS COLOUR" ("Enum")) -> (s? t:f=w2568:u16)
                n844 = Select(t=w2568, s=w2566, f=State_Type_Definitions,_for_0.26d_versions_and_later."Task 9N: SCAN IMAGE" ("Enum")) -> (s? t:f=w2574:u16)
              }
              frame "Exit" {
                n845 = for {
                  shift-right: [w2593] -> w2590
                  shift-left: w2587 -> [w2594]
                  tunnel: string[] ["STOP", "RESET ENCODERS", "RESET YAW", ""] -> [w2592] mode=indexing
                  n846 = Enqueue Element(queue=w2594, element=w2592) -> (queue out=w2593:refnum<queue>)  [unwired: 2 in, 2 out]
                }
              }
            }
          }
          frame 52 {
            # ">> Item Selection Bias >>"
            n847 = Dequeue Element(queue=w2602, timeout in ms (-1)=w2601, error in (no error)=w2600) -> (element=w2604:T10)  [unwired: 3 out]
            n848 = case shown="\"Start Task 1\", Default" w2604 {
              tunnel: w2595 -> [w2610 _]
              tunnel: [w2617 State_Type_Definitions,_for_0.26g_versions_and_later_2."True Stop" ("Enum")] -> w2598
              tunnel: w2599 -> [w2609 _]
              tunnel: w2603 -> [w2616 w2633]
              tunnel: [w2615 w2634] -> w2597
              tunnel: [State_Type_Definitions,_for_0.26g_versions_and_later_2."Idle" ("Enum") State_Type_Definitions,_for_0.26g_versions_and_later_2."Shutdown" ("Enum")] -> w2596
              frame "Start Task 1", Default {
                n849 = case shown="False" w2610 {
                  tunnel: w2616 -> [w2620 w2627]
                  tunnel: [w2621 w2626] -> w2615
                  frame False {
                    n850 = for {
                      tunnel: string[] ["START TIMER", "COLOUR PROCESSING", ""] ("element") -> [w2622] mode=indexing
                      shift-right: [w2624] -> w2621
                      shift-left: w2620 -> [w2623]
                      n851 = Enqueue Element(queue=w2623, element=w2622) -> (queue out=w2624:refnum<queue>)  [unwired: 2 in, 2 out]
                    }
                  }
                  frame True {
                    n852 = for {
                      shift-right: [w2629] -> w2626
                      shift-left: w2627 -> [w2630]
                      tunnel: string[] ["CLOSE CAM", "DISPOSE BUFFERS", "RESET ENCODERS", "RESET YAW", "RESET FLAGS", ""] -> [w2628] mode=indexing
                      n853 = Enqueue Element(queue=w2630, element=w2628) -> (queue out=w2629:refnum<queue>)  [unwired: 2 in, 2 out]
                    }
                  }
                }
                n854 = Or(x=w2610, y=w2609) -> (x .or. y?=w2608:bool)
                n855 = Select(t=State_Type_Definitions,_for_0.26g_versions_and_later_2."True Stop" ("Enum"), s=w2609, f=State_Type_Definitions,_for_0.26d_versions_and_later."Task 9P: MOVE RIGHT" ("Enum")) -> (s? t:f=w2611:u16)
                n856 = Select(t=w2611, s=w2608, f=State_Type_Definitions,_for_0.26d_versions_and_later."Task 9O: PROCESS COLOUR" ("Enum")) -> (s? t:f=w2617:u16)
              }
              frame "Exit" {
                n857 = for {
                  shift-right: [w2637] -> w2634
                  shift-left: w2633 -> [w2638]
                  tunnel: string[] ["STOP", "RESET ENCODERS", "RESET YAW", "ARDUINO MODE 0"] -> [w2636] mode=indexing
                  n858 = Enqueue Element(queue=w2638, element=w2636) -> (queue out=w2637:refnum<queue>)  [unwired: 2 in, 2 out]
                }
              }
            }
          }
          frame 53 {
            # ">> Item Selection Bias >>"
            n859 = Dequeue Element(queue=w2644, timeout in ms (-1)=w2643, error in (no error)=w2642) -> (element=w2652:T10)  [unwired: 3 out]
            n860 = Greater?(x=w2640, y=50.0) -> (0:w2650:bool)
            n861 = And(x=w2639, y=w2650) -> (x .and. y?=w2651:bool)
            n862 = case shown="\"Start Task 1\", Default" w2652 {
              tunnel: w2651 -> [w2658 _]
              tunnel: [w2665 State_Type_Definitions,_for_0.26g_versions_and_later_2."True Stop" ("Enum")] -> w2647
              tunnel: w2641 -> [w2657 _]
              tunnel: w2645 -> [w2664 w2681]
              tunnel: [w2663 w2682] -> w2646
              tunnel: [State_Type_Definitions,_for_0.26g_versions_and_later_2."Idle" ("Enum") State_Type_Definitions,_for_0.26g_versions_and_later_2."Shutdown" ("Enum")] -> w2648
              frame "Start Task 1", Default {
                n863 = case shown="False" w2658 {
                  tunnel: w2664 -> [w2668 w2675]
                  tunnel: [w2669 w2674] -> w2663
                  frame False {
                    n864 = for {
                      tunnel: string[] ["READ LINE SENSOR", "READ NAVX", "RIGHT", "READ ENCODERS"] ("element") -> [w2670] mode=indexing
                      shift-right: [w2672] -> w2669
                      shift-left: w2668 -> [w2671]
                      n865 = Enqueue Element(queue=w2671, element=w2670) -> (queue out=w2672:refnum<queue>)  [unwired: 2 in, 2 out]
                    }
                  }